vi "真正主程序.vi"() -> ()   [LabVIEW 2013]
doc: "该模板用于创建生产者／消费者模式的应用程序，以事件驱动的方式，生成队列中的项。如需通过响应事件实现代码的异步执行，同时不影响用户界面的响应速度，可考虑用该模式替代“用户界面事件处理器”模式。"
panel:
  in  "战斗失败":bool
  out "怪物血值":i32=380
  in  "战斗胜利":bool
  out "五个状态 2":enum16{"神不足", "逃跑", "初始化", "物品", "仙术", "攻击"}(ring)=enum."逃跑"
  in  "神值不够":bool
  in  "逃跑成功":bool
  out "沈欺霜 2":i32(slide) scale=0.0..200.0
  in  "龙蟠雕玉":cluster{"琉璃法珠":bool, "介绍框":bool, "剩余":dbl}
  in  "疾风术簇":T1
  in  "凝冰术簇":T2
  in  "火爪术簇":T3
  in  "普通攻击簇":T4
  out "集气攻击待机动作":bool
  in  "集气攻击簇":T5
  in  "怪物":bool=TRUE
  in  "确定按敌人攻击值钮":bool
  in  "怪兽 2":bool=TRUE
  in  "怪物状态":enum16{"初始化", "后退", "施法", "出击"}(ring)
  in  "枚举":enum16{"我方攻击", "敌人战斗", "时间条"}(ring)
  in  "主控":enum16{"我方攻击", "敌方攻击", "时间条", ""}(ring)
  out "怪物行走":i32(slide)=64 scale=0.0..100.0
  out "人物行走":i32(slide)=105 scale=0.0..100.0
  in  "待机":bool
  out "神":i32(slide)=150 scale=0.0..200.0
  out "沈欺霜":i32(slide)=150 scale=0.0..200.0
  in  "琉璃法珠簇":cluster{"琉璃法珠":bool, "介绍框":bool, "剩余":dbl}
  in  "仙术簇":T6={"火爪术"=TRUE, "凝冰术"=FALSE, "疾风术"=FALSE, "仙术中的放弃"=TRUE}
  in  "物品簇":cluster{"止血草":bool, "鼠儿果":bool, "物品中的放弃":bool}={"止血草"=FALSE, "鼠儿果"=FALSE, "物品中的放弃"=TRUE}
  in  "攻击簇":cluster{"普通攻击":bool, "集气攻击":bool, "攻击中的放弃":bool}={"普通攻击"=TRUE, "集气攻击"=FALSE, "攻击中的放弃"=FALSE}
  in  "逃跑":bool
  in  "物品":bool
  in  "仙术":bool
  in  "攻击":bool
  in  "五个状态":enum16{"逃跑", "初始化", "物品", "仙术", "攻击"}(ring)
  in  "怪兽":bool
  # "框图坐标\n207,421,460，498\n沈欺霜坐标\n800,388"
  # "剩余"
  # "个"
  # "剩余"
  # "个"
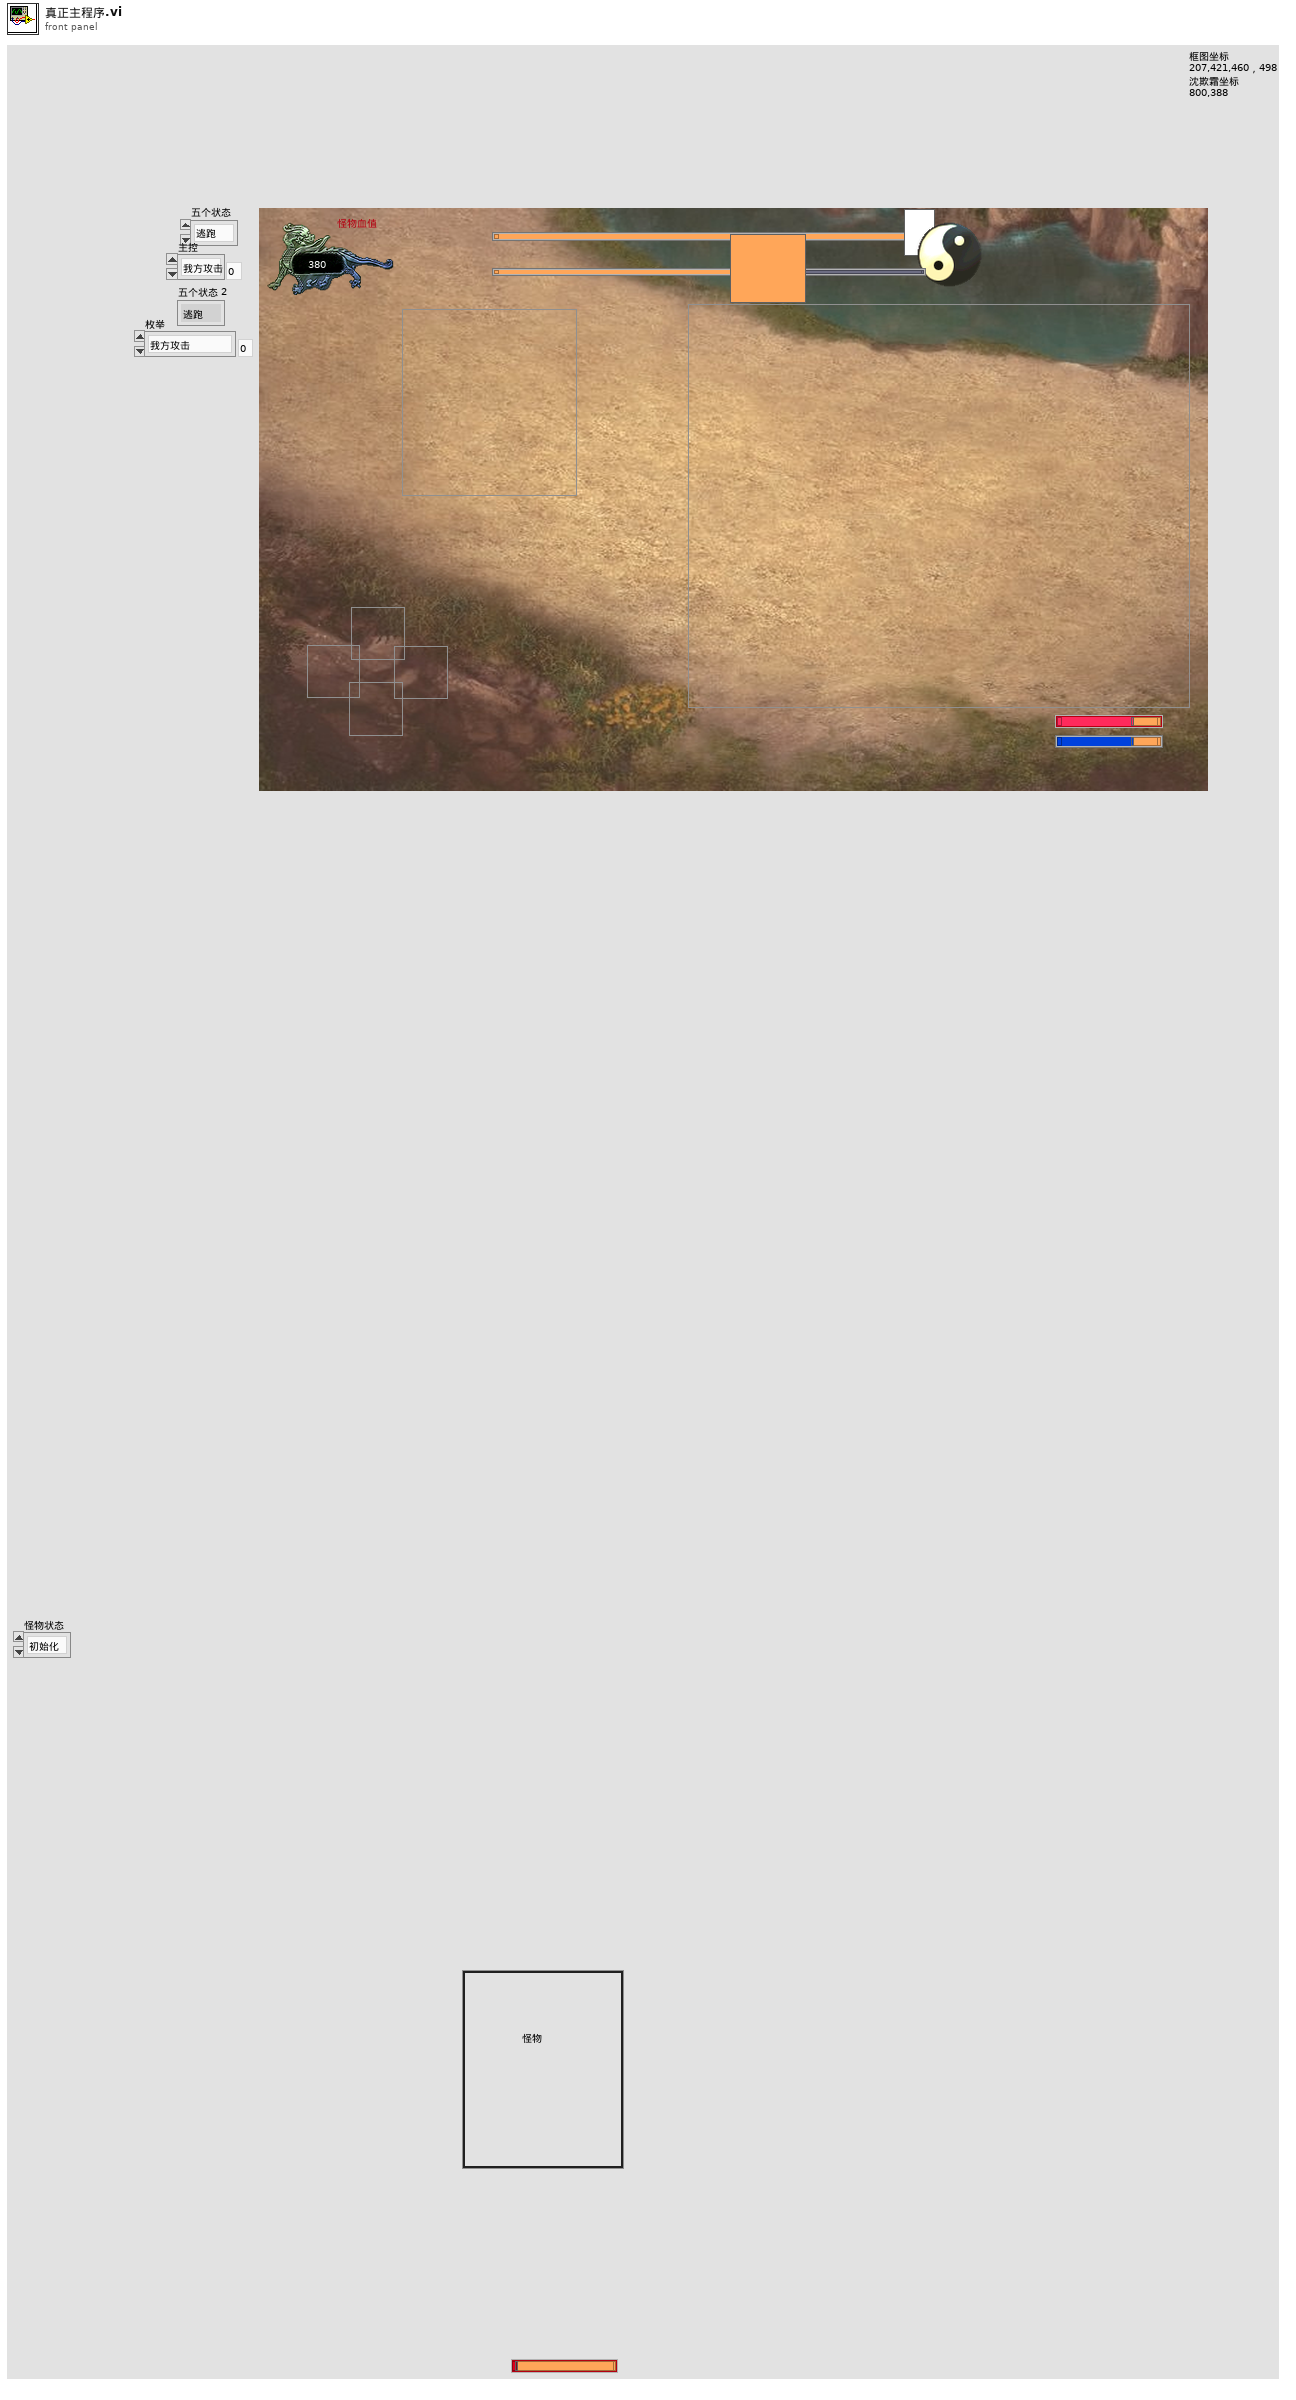
[diagram p1: front panel]
types:
  T1 = cluster{"确定按钮":bool, "确定按钮 2":bool, "确定按钮 3":bool, "确定按钮 4":bool, "确定按钮 5":bool, "确定按钮 6":bool, "确定按钮 7":bool, "确定按钮 8":bool, "确定按钮 9":bool, "确定按钮 10":bool, "确定按钮 11":bool, "确定按钮 12":bool, "确定按钮 13":bool, "确定按钮 14":bool, "确定按钮 15":bool}
  T2 = cluster{"确定按钮1":bool, "确定按钮 2":bool, "确定按钮 3":bool, "确定按钮 4":bool, "确定按钮 5":bool, "确定按钮 6":bool, "确定按钮 7":bool, "确定按钮 8":bool, "确定按钮 9":bool, "确定按钮 10":bool, "确定按钮 11":bool, "确定按钮 12":bool, "确定按钮 13":bool, "确定按钮 14":bool, "确定按钮 15":bool, bool}
  T3 = cluster{"4":bool, "5":bool, "6":bool, "7":bool, "8":bool, "1":bool, "2":bool, "3":bool, "9":bool, "10":bool, "11":bool, "12":bool, "13":bool, "14":bool, "15":bool, "确定按钮":bool}
  T4 = cluster{"1":bool, "2":bool, "3":bool, "4":bool, "5":bool, "6":bool, "7":bool, "8":bool, "9":bool, "减50":bool}
  T5 = cluster{"1":bool, "2":bool, "3":bool, "4":bool, "5":bool, "6":bool, "7":bool, "8":bool, "9":bool, "10":bool, "11":bool, "12":bool, "13":bool, "14":bool, "15":bool, "16":bool, "17":bool}
  T6 = cluster{"火爪术":bool, "凝冰术":bool, "疾风术":bool, "仙术中的放弃":bool}
  T7 = cluster{"1":bool, "2":bool, "3":bool, "4":bool, "5":bool, "6":bool, "7":bool, "8":bool, "9":bool}
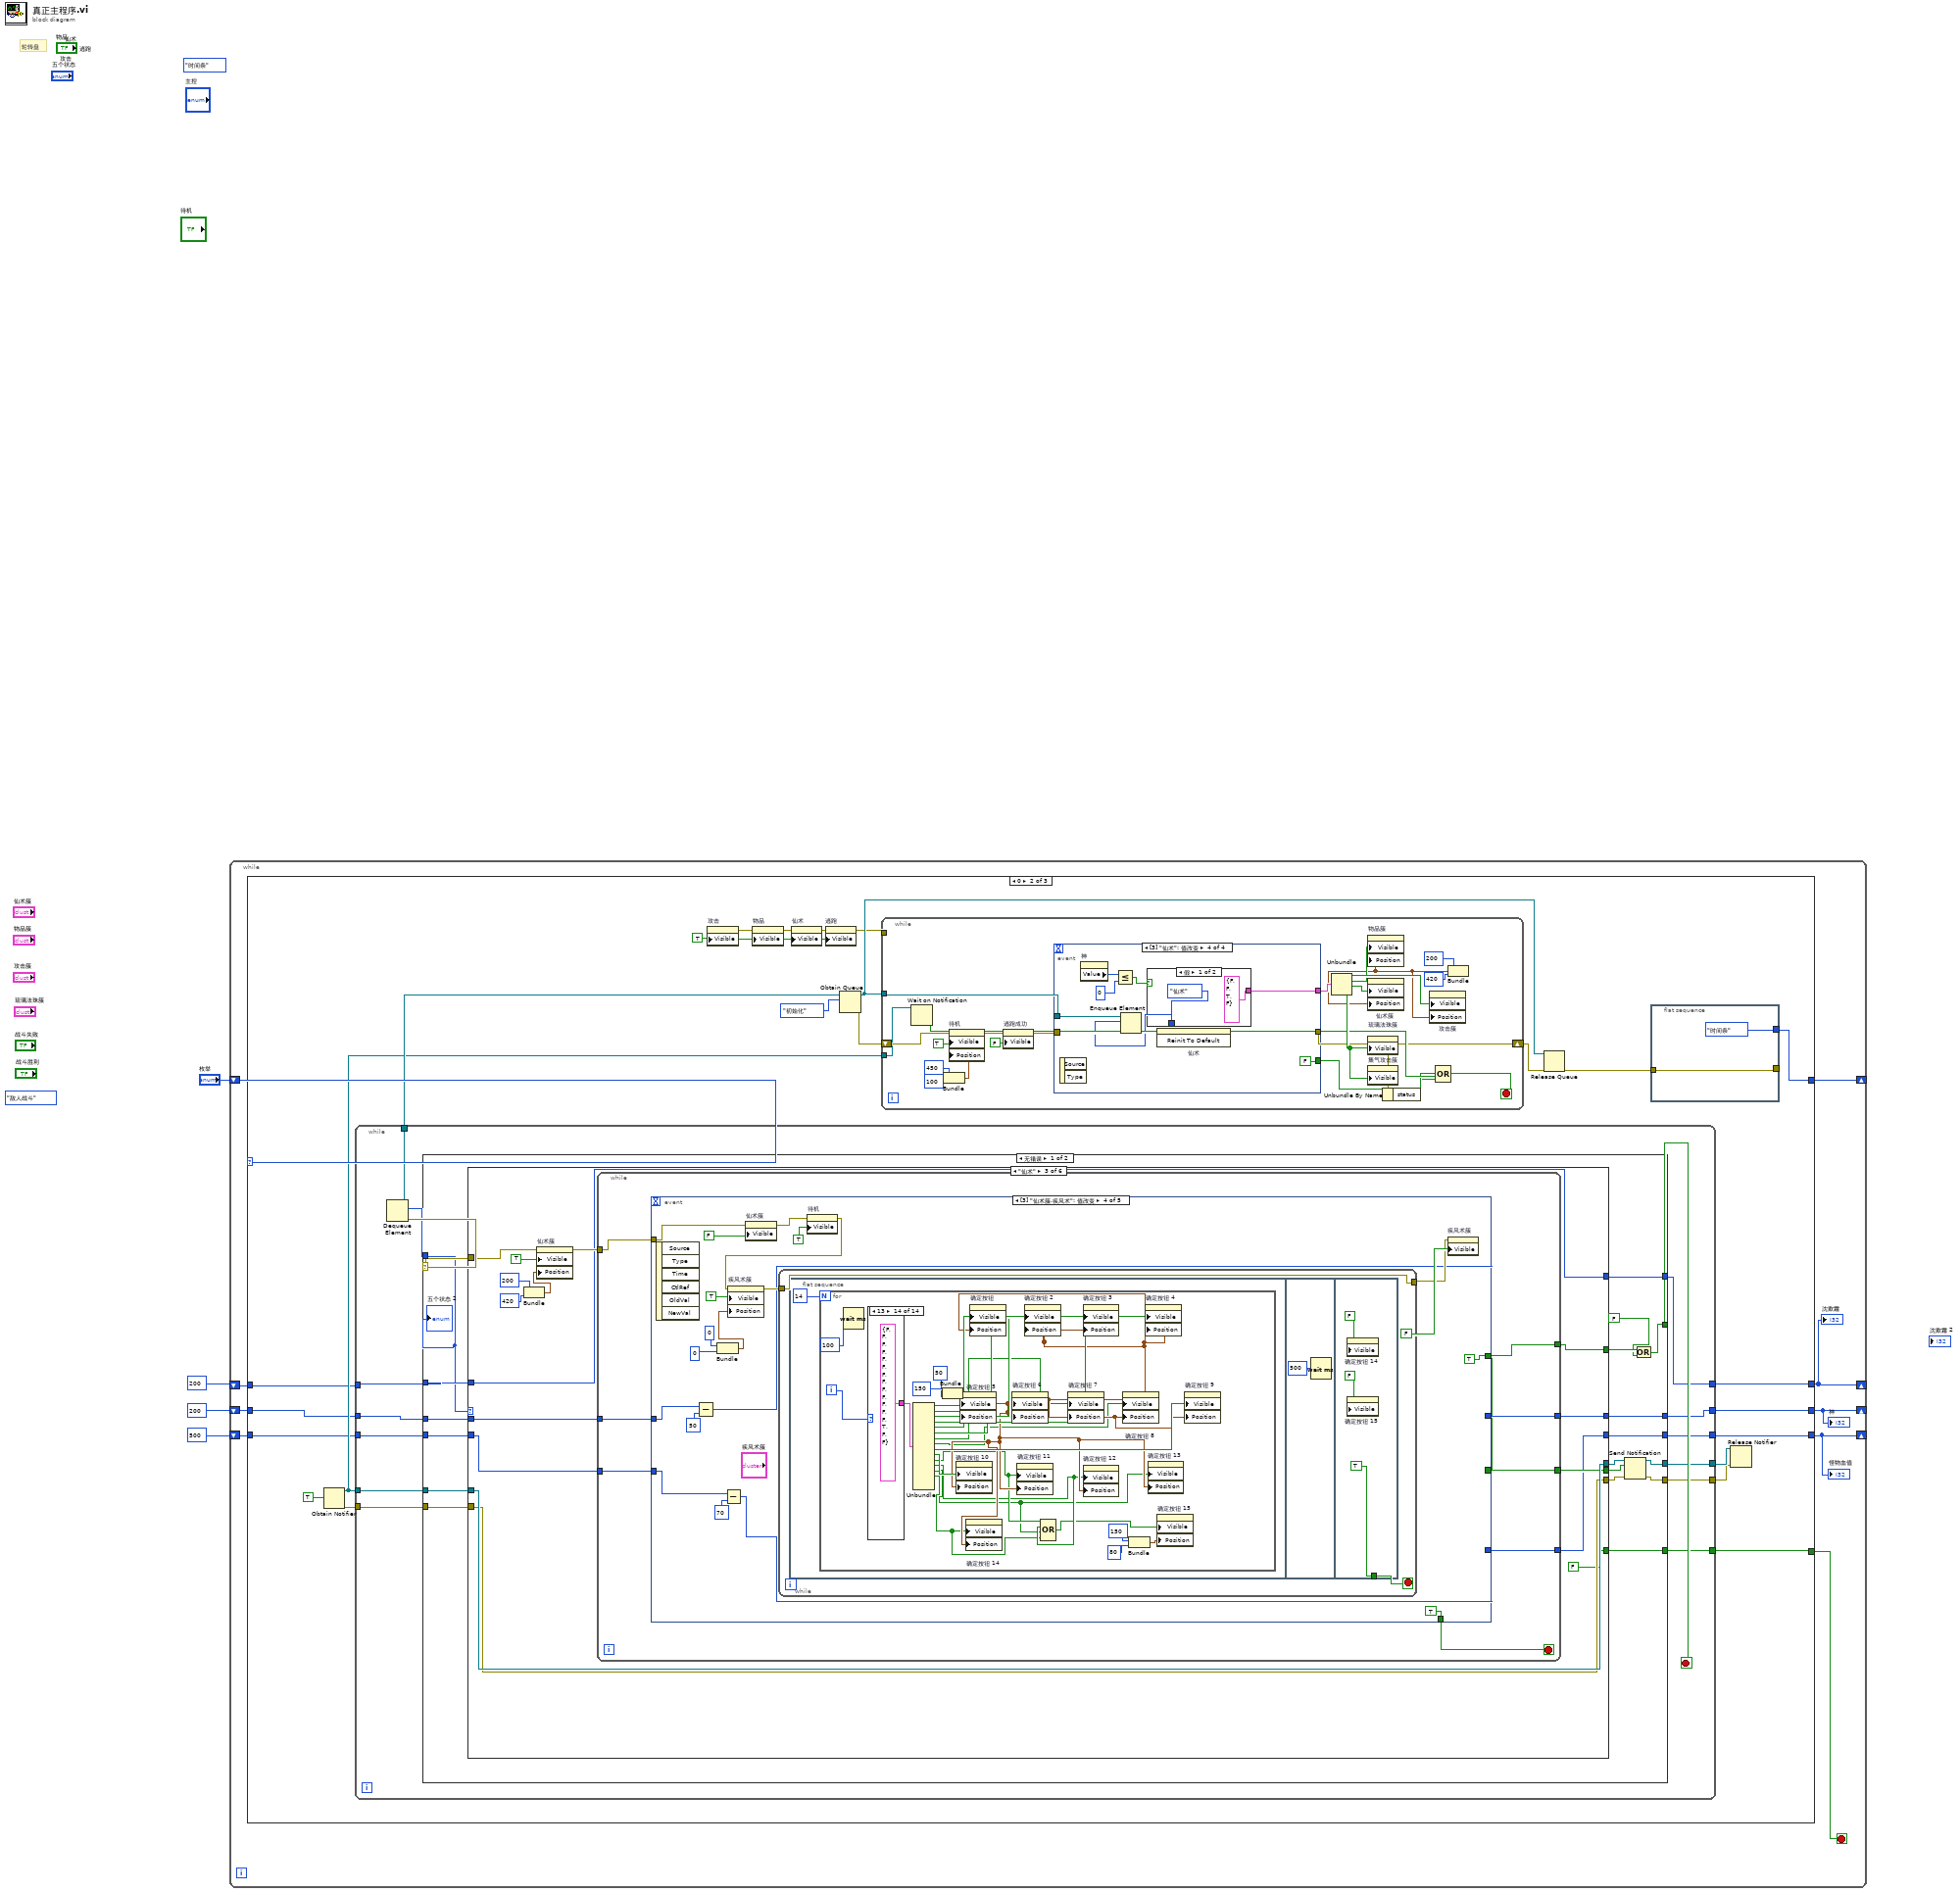
[diagram p0: block diagram]
diagram:
  (unwired) enum16{"我方攻击", "敌人战斗", "时间条"}."敌人战斗" ("枚举")
  (unwired) enum16{"我方攻击", "敌方攻击", "时间条", ""}."时间条" ("主控")
  # "轮转盘"
  n1 = while {
    shift-right: [w12] -> _
    shift-left: "枚举" -> [w13]
    shift-right: [w8] -> _
    shift-left: 200 -> [w11]
    shift-right: [w9] -> _
    shift-left: 200 -> [w10]
    shift-right: [w5] -> _
    shift-left: 500 -> [w7]
    stop <- w6 stop-if-true
    n2 = case shown="0" w13 {
      tunnel: [enum16{"我方攻击", "敌方攻击", "时间条", ""}."时间条" ("主控") w132 w790] -> w12
      tunnel: w11 -> [w22 w121 w784]
      tunnel: w10 -> [w21 w120 w789]
      tunnel: [w15 w119 w784] -> w8
      tunnel: [w21 w118 w789] -> w9
      tunnel: w7 -> [w20 w115 w786]
      tunnel: [w20 w114 w786] -> w5
      tunnel: [w17 w113 w785] -> w6
      frame 1 {
        w28 = FALSE
        n3 = Subtract(x=w22, y=50) -> (x-y=w16:i32)
        n4 = property on="攻击" class="Bool"("Visible"=w28) -> (error out=w27:errorcluster)  [unwired: 2 in, 1 out]
        n5 = property on="逃跑" class="Bool"(error in=w27, "Visible"=w28) -> (error out=w26:errorcluster)  [unwired: 1 in, 1 out]
        n6 = property on="物品" class="Bool"(error in=w26, "Visible"=w28) -> (error out=w25:errorcluster)  [unwired: 1 in, 1 out]
        n7 = property on="仙术" class="Bool"(error in=w25, "Visible"=w28) -> (error out=w24:errorcluster)  [unwired: 1 in, 1 out]
        n8 = while {
          shift-right: [w41] -> _
          shift-left: "怪物状态" -> [w43]
          tunnel: [w42] -> w14
          tunnel: w24 -> [_]
          stop <- w40 stop-if-true
          # "敌人攻击"
          n9 = case shown="\"后退\"" w43 {
            tunnel: [FALSE TRUE FALSE] -> w40
            tunnel: [w49 w61 w91] -> w42
            tunnel: [enum16{"初始化", "后退", "施法", "出击"}."出击" ("枚举") enum16{"初始化", "后退", "施法", "出击"}."初始化" ("枚举 2") enum16{"初始化", "后退", "施法", "出击"}."后退" ("枚举")] -> w41
            frame "初始化", Default {
              n10 = Bundle(550, 200) -> (w53:cluster{i32, i32})  [unwired: 1 in]
              n11 = Bundle(150, 100) -> (w54:cluster{i32, i32})  [unwired: 1 in]
              n12 = property on="怪兽" class="Bool"("Visible"=TRUE, "Position"=w54) -> (error out=w50:errorcluster)  [unwired: 2 in, 1 out]
              n13 = property on="怪兽 2" class="Bool"(error in=w50, "Visible"=FALSE, "Position"=w53) -> (error out=w49:errorcluster)  [unwired: 1 in, 1 out]
            }
            frame "后退" {
              n14 = property on="怪兽" class="Bool"("Visible"=FALSE) -> (error out=w59:errorcluster)  [unwired: 2 in, 1 out]
              n15 = for {
                N: 20 -> [_]
                tunnel: w59 -> [w76]
                tunnel: [w75] -> w63
                i -> [w73]
                n16 = Multiply(x=20, y=w73) -> (x*y=w77:i32)
                n17 = Subtract(x=550, y=w77) -> (x-y=w74:i32)
                n18 = Multiply(x=5, y=w73) -> (x*y=w71:i32)
                n19 = Wait (ms)(milliseconds to wait=u32 10 ("等待时间（毫秒）")) -> ()  [unwired: 1 out]
                n20 = Subtract(x=200, y=w71) -> (x-y=w69:i32)
                n21 = Bundle(w74, w69) -> (w80:cluster{i32, i32})  [unwired: 1 in]
                n22 = property on="怪兽 2" class="Bool"(error in=w76, "Visible"=TRUE, "Position"=w80) -> (error out=w75:errorcluster)  [unwired: 1 in, 1 out]
              }
              n23 = Bundle(150, 100) -> (w65:cluster{i32, i32})  [unwired: 1 in]
              n24 = property on="怪兽 2" class="Bool"(error in=w63, "Visible"=FALSE) -> (error out=w62:errorcluster)  [unwired: 1 in, 1 out]
              n25 = property on="怪兽" class="Bool"(error in=w62, "Visible"=TRUE, "Position"=w65) -> (error out=w61:errorcluster)  [unwired: 1 in, 1 out]
            }
            frame "出击" {
              n26 = for {
                N: 20 -> [_]
                tunnel: [w109] -> w94
                tunnel: [w102] -> w90
                tunnel: [w101] -> w86
                i -> [w107]
                n27 = Multiply(x=w107, y=20) -> (x*y=w101:i32)
                n28 = Add(x=150, y=w101) -> (x+y=w103:i32)
                n29 = Multiply(x=w107, y=5) -> (x*y=w106:i32)
                n30 = Wait (ms)(milliseconds to wait=u32 1 ("等待时间（毫秒）")) -> ()  [unwired: 1 out]
                n31 = Add(x=100, y=w106) -> (x+y=w102:i32)
                n32 = Bundle(w103, w102) -> (w111:cluster{i32, i32})  [unwired: 1 in]
                n33 = property on="怪兽" class="Bool"("Position"=w111) -> (error out=w109:errorcluster)  [unwired: 2 in, 1 out]
              }
              n34 = Subtract(x=w90, y=60) -> (x-y=w88:i32)
              n35 = Add(x=w86, y=300) -> (x+y=w85:i32)
              n36 = Bundle(w85, w88) -> (w84:cluster{i32, i32})  [unwired: 1 in]
              n37 = property on="确定按敌人攻击值钮" class="Bool"(error in=w94, "Visible"=TRUE, "Position"=w84) -> (error out=w93:errorcluster)  [unwired: 1 in, 1 out]
              n38 = flat-sequence {
                tunnel: w93 -> [w99]
                tunnel: [w99] -> _
                tunnel: [w99] -> w92
                frame #0 {
                  n39 = Wait (ms)(milliseconds to wait=500) -> ()  [unwired: 1 out]
                }
              }
              n40 = property on="确定按敌人攻击值钮" class="Bool"(error in=w92, "Visible"=FALSE) -> (error out=w91:errorcluster)  [unwired: 1 in, 1 out]
            }
          }
        }
        n41 = Less Or Equal?(x=w16, y=0) -> (x <= y?=w18:bool)
        n42 = case shown="假" w18 {
          tunnel: [FALSE w38] -> w17
          tunnel: w16 -> [w32 w39]
          tunnel: [w32 w39] -> w15
          tunnel: w14 -> [w31 w34]
          tunnel: [w31 w34] -> _
          frame False {
          }
          frame True {
            w38 = TRUE
            n43 = Bundle(200, 200) -> (w35:cluster{i32, i32})  [unwired: 1 in]
            n44 = property on="战斗失败" class="Bool"("Visible"=w38, "Position"=w35) -> ()  [unwired: 2 in, 2 out]
          }
        }
      }
      frame 0 {
        w123 = TRUE
        n45 = Obtain Notifier(notification data type=TRUE) -> (notifier out=w127:refnum<notifier>, error out=w128:errorcluster)  [unwired: 3 in, 1 out]
        n46 = property on="攻击" class="Bool"("Visible"=w123) -> (error out=w126:errorcluster)  [unwired: 2 in, 1 out]
        n47 = property on="物品" class="Bool"(error in=w126, "Visible"=w123) -> (error out=w125:errorcluster)  [unwired: 1 in, 1 out]
        n48 = property on="仙术" class="Bool"(error in=w125, "Visible"=w123) -> (error out=w124:errorcluster)  [unwired: 1 in, 1 out]
        n49 = property on="逃跑" class="Bool"(error in=w124, "Visible"=w123) -> (error out=w122:errorcluster)  [unwired: 1 in, 1 out]
        n50 = Obtain Queue(element data type=enum16{"神不足", "逃跑", "初始化", "物品", "仙术", "攻击"}."初始化" ("五个状态")) -> (queue out=w134:refnum<queue>, error out=w135:errorcluster)  [unwired: 4 in, 1 out]
        n51 = while {
          tunnel: w134 -> [w149]
          tunnel: w127 -> [w148]
          tunnel: [w147] -> w130
          tunnel: [w146] -> w129
          tunnel: w128 -> [w145]
          tunnel: w121 -> [w144]
          tunnel: w120 -> [w143]
          tunnel: [w142] -> w119
          tunnel: [w141] -> w118
          tunnel: w115 -> [w140]
          tunnel: [w139] -> w114
          tunnel: [w138] -> w113
          stop <- w150 stop-if-true
          n52 = Dequeue Element(queue=w149) -> (element=w151:enum16{"神不足", "逃跑", "初始化", "物品", "仙术", "攻击"}, error out=w152:errorcluster)  [unwired: 2 in, 2 out]
          n53 = case shown="无错误" w152 {
            selector: w152 -> [w171 _]
            tunnel: w151 -> [w156 _]
            tunnel: [w164 TRUE] -> w150
            tunnel: w144 -> [w170 w719]
            tunnel: [w169 w719] -> w142
            tunnel: w143 -> [w168 w718]
            tunnel: [w167 w718] -> w141
            tunnel: w148 -> [w163 w717]
            tunnel: [w157 w717] -> w147
            tunnel: [w158 w716] -> w146
            tunnel: w145 -> [w162 w716]
            tunnel: w140 -> [w155 w715]
            tunnel: [w154 w715] -> w139
            tunnel: [w153 TRUE] -> w138
            frame No Error {
              n54 = case shown="\"仙术\"" w156 {
                tunnel: w171 -> [_ w196 w366 w605 w690 _]
                tunnel: w170 -> [w179 w190 w364 w600 w689 w709]
                tunnel: [w179 w190 w364 w599 w689 w709] -> w169
                tunnel: w168 -> [w178 w189 w359 w594 w688 w708]
                tunnel: [w178 w189 w358 w593 w688 w708] -> w167
                tunnel: [FALSE w188 w363 w588 w683 FALSE] -> w166
                tunnel: w163 -> [w176 w187 w362 w590 w682 w705]
                tunnel: [w176 w185 w362 w590 w682 w705] -> w161
                tunnel: [w175 w183 w361 w589 w681 w704] -> w159
                tunnel: w162 -> [w175 w186 w361 w589 w681 w704]
                tunnel: [FALSE w184 w360 w588 TRUE FALSE] -> w160
                tunnel: w155 -> [w173 w182 w357 w587 w679 w696]
                tunnel: [w173 w181 w356 w587 w679 w696] -> w154
                tunnel: [FALSE FALSE FALSE FALSE TRUE FALSE] -> w153
                frame "初始化", Default {
                }
                frame "攻击" {
                  n55 = Bundle(200, 420) -> (w191:cluster{i32, i32})  [unwired: 1 in]
                  n56 = property on="攻击簇" class="Clust"(error in=w196, "Visible"=TRUE, "Position"=w191) -> (error out=w194:errorcluster)  [unwired: 1 in, 1 out]
                  n57 = while {
                    tunnel: w194 -> [w206]
                    tunnel: [w203] -> w188
                    tunnel: w187 -> [w202]
                    tunnel: w186 -> [w199]
                    tunnel: [w201] -> w185
                    tunnel: [w200] -> w184
                    tunnel: [w199] -> w183
                    tunnel: w182 -> [w198]
                    tunnel: [w197] -> w181
                    stop <- w207 stop-if-true
                    n58 = event shown="[3] \"攻击簇.普通攻击\": 值改变" {
                      selector: _ -> [_ _ _ _]
                      dyn-events: _ -> [_ _ _ _]
                      timeout: _ -> [_ _ _ _]
                      tunnel: [w210 w217 w299 w307] -> w205
                      tunnel: [FALSE TRUE TRUE TRUE] -> w207
                      tunnel: w206 -> [w210 w223 w299 w319]
                      tunnel: [w209 w215 w297 w305] -> w203
                      tunnel: w202 -> [w208 w216 w298 w304]
                      tunnel: [w208 w216 w298 w304] -> w201
                      tunnel: [w209 w215 w297 w305] -> w200
                      tunnel: w198 -> [_ w213 w296 w302]
                      tunnel: [_ w212 w296 w301] -> w197
                      event Timeout {
                        w209 = FALSE
                        n59 = event-data() -> ()  [unwired: 1 in, 3 out]
                      }
                      event "攻击簇.集气攻击": Value Change {
                        w215 = TRUE
                        w232 = TRUE ("可见")
                        n60 = event-data() -> ()  [unwired: 1 in, 6 out]
                        n61 = Bundle(450, 100) -> (w237:cluster{i32, i32})  [unwired: 1 in]
                        n62 = property on="待机" class="Bool"(error in=w223, "Visible"=FALSE) -> (error out=w224:errorcluster)  [unwired: 1 in, 1 out]
                        n63 = property on="攻击簇" class="Clust"(error in=w224, "Visible"=FALSE) -> (error out=w231:errorcluster)  [unwired: 1 in, 1 out]
                        n64 = property on="集气攻击待机动作" class="Bool"(error in=w231, "Position"=w237, "Visible"=w232) -> (error out=w240:errorcluster)  [unwired: 1 in, 1 out]
                        n65 = property on="集气攻击簇" class="Clust"(error in=w231, "Visible"=w232) -> (error out=w230:errorcluster)  [unwired: 1 in, 1 out]
                        n66 = Subtract(x=w213, y=100) -> (x-y=w212:i32)
                        n67 = for {
                          N: 20 -> [_]
                          shift-right: [w288] -> _
                          shift-left: _ -> [_]
                          tunnel: w240 -> [w289]
                          tunnel: [w289] -> w235
                          i -> [w290]
                          n68 = Quotient & Remainder(x=w290, y=2) -> (x-y*floor(x/y)=w292:i32)  [unwired: 1 out]
                          n69 = case shown="1" w292 {
                            tunnel: [TRUE FALSE] -> w288
                            frame 0, Default {
                            }
                            frame 1 {
                            }
                          }
                          "集气攻击待机动作" <- w288
                          n70 = Wait (ms)(milliseconds to wait=u32 100 ("等待时间（毫秒）")) -> ()  [unwired: 1 out]
                        }
                        n71 = while {
                          tunnel: w230 -> [w242]
                          tunnel: [w242] -> w229
                          stop <- w243 stop-if-true
                          n72 = flat-sequence {
                            tunnel: [TRUE] -> w243
                            frame #0 {
                              n73 = for {
                                N: 17 -> [_]
                                i -> [w256]
                                n74 = Wait (ms)(milliseconds to wait=100) -> ()  [unwired: 1 out]
                                n75 = case shown="0, 默认" w256 {
                                tunnel: [T5 {"1"=TRUE, "2"=FALSE, "3"=FALSE, "4"=FALSE, "5"=FALSE, "6"=FALSE, "7"=FALSE, "8"=FALSE, "9"=FALSE, "10"=FALSE, "11"=FALSE, "12"=FALSE, "13"=FALSE, "14"=FALSE, "15"=FALSE, "16"=FALSE, "17"=FALSE} ("簇") T5 {"1"=FALSE, "2"=TRUE, "3"=FALSE, "4"=FALSE, "5"=FALSE, "6"=FALSE, "7"=FALSE, "8"=FALSE, "9"=FALSE, "10"=FALSE, "11"=FALSE, "12"=FALSE, "13"=FALSE, "14"=FALSE, "15"=FALSE, "16"=FALSE, "17"=FALSE} ("簇") T5 {"1"=FALSE, "2"=FALSE, "3"=TRUE, "4"=FALSE, "5"=FALSE, "6"=FALSE, "7"=FALSE, "8"=FALSE, "9"=FALSE, "10"=FALSE, "11"=FALSE, "12"=FALSE, "13"=FALSE, "14"=FALSE, "15"=FALSE, "16"=FALSE, "17"=FALSE} ("簇") T5 {"1"=FALSE, "2"=FALSE, "3"=FALSE, "4"=TRUE, "5"=FALSE, "6"=FALSE, "7"=FALSE, "8"=FALSE, "9"=FALSE, "10"=FALSE, "11"=FALSE, "12"=FALSE, "13"=FALSE, "14"=FALSE, "15"=FALSE, "16"=FALSE, "17"=FALSE} ("簇") T5 {"1"=FALSE, "2"=FALSE, "3"=FALSE, "4"=FALSE, "5"=TRUE, "6"=FALSE, "7"=FALSE, "8"=FALSE, "9"=FALSE, "10"=FALSE, "11"=FALSE, "12"=FALSE, "13"=FALSE, "14"=FALSE, "15"=FALSE, "16"=FALSE, "17"=FALSE} ("簇") T5 {"1"=FALSE, "2"=FALSE, "3"=FALSE, "4"=FALSE, "5"=FALSE, "6"=TRUE, "7"=FALSE, "8"=FALSE, "9"=FALSE, "10"=FALSE, "11"=FALSE, "12"=FALSE, "13"=FALSE, "14"=FALSE, "15"=FALSE, "16"=FALSE, "17"=FALSE} ("簇") T5 {"1"=FALSE, "2"=FALSE, "3"=FALSE, "4"=FALSE, "5"=FALSE, "6"=FALSE, "7"=TRUE, "8"=FALSE, "9"=FALSE, "10"=FALSE, "11"=FALSE, "12"=FALSE, "13"=FALSE, "14"=FALSE, "15"=FALSE, "16"=FALSE, "17"=FALSE} ("簇") T5 {"1"=FALSE, "2"=FALSE, "3"=FALSE, "4"=FALSE, "5"=FALSE, "6"=FALSE, "7"=FALSE, "8"=TRUE, "9"=FALSE, "10"=FALSE, "11"=FALSE, "12"=FALSE, "13"=FALSE, "14"=FALSE, "15"=FALSE, "16"=FALSE, "17"=FALSE} ("簇") T5 {"1"=FALSE, "2"=FALSE, "3"=FALSE, "4"=FALSE, "5"=FALSE, "6"=FALSE, "7"=FALSE, "8"=FALSE, "9"=TRUE, "10"=FALSE, "11"=FALSE, "12"=FALSE, "13"=FALSE, "14"=FALSE, "15"=FALSE, "16"=FALSE, "17"=FALSE} ("簇") T5 {"1"=FALSE, "2"=FALSE, "3"=FALSE, "4"=FALSE, "5"=FALSE, "6"=FALSE, "7"=FALSE, "8"=FALSE, "9"=FALSE, "10"=TRUE, "11"=FALSE, "12"=FALSE, "13"=FALSE, "14"=FALSE, "15"=FALSE, "16"=FALSE, "17"=FALSE} ("簇") T5 {"1"=FALSE, "2"=FALSE, "3"=FALSE, "4"=FALSE, "5"=FALSE, "6"=FALSE, "7"=FALSE, "8"=FALSE, "9"=FALSE, "10"=FALSE, "11"=TRUE, "12"=FALSE, "13"=FALSE, "14"=FALSE, "15"=FALSE, "16"=FALSE, "17"=FALSE} ("簇") T5 {"1"=FALSE, "2"=FALSE, "3"=FALSE, "4"=FALSE, "5"=FALSE, "6"=FALSE, "7"=FALSE, "8"=FALSE, "9"=FALSE, "10"=FALSE, "11"=FALSE, "12"=TRUE, "13"=FALSE, "14"=FALSE, "15"=FALSE, "16"=FALSE, "17"=FALSE} ("簇") T5 {"1"=FALSE, "2"=FALSE, "3"=FALSE, "4"=FALSE, "5"=FALSE, "6"=FALSE, "7"=FALSE, "8"=FALSE, "9"=FALSE, "10"=FALSE, "11"=FALSE, "12"=FALSE, "13"=TRUE, "14"=FALSE, "15"=FALSE, "16"=FALSE, "17"=FALSE} ("簇") T5 {"1"=FALSE, "2"=FALSE, "3"=FALSE, "4"=FALSE, "5"=FALSE, "6"=FALSE, "7"=FALSE, "8"=FALSE, "9"=FALSE, "10"=FALSE, "11"=FALSE, "12"=FALSE, "13"=FALSE, "14"=TRUE, "15"=FALSE, "16"=FALSE, "17"=FALSE} ("簇") T5 {"1"=FALSE, "2"=FALSE, "3"=FALSE, "4"=FALSE, "5"=FALSE, "6"=FALSE, "7"=FALSE, "8"=FALSE, "9"=FALSE, "10"=FALSE, "11"=FALSE, "12"=FALSE, "13"=FALSE, "14"=FALSE, "15"=TRUE, "16"=FALSE, "17"=FALSE} ("簇") T5 {"1"=FALSE, "2"=FALSE, "3"=FALSE, "4"=FALSE, "5"=FALSE, "6"=FALSE, "7"=FALSE, "8"=FALSE, "9"=FALSE, "10"=FALSE, "11"=FALSE, "12"=FALSE, "13"=FALSE, "14"=FALSE, "15"=FALSE, "16"=TRUE, "17"=FALSE} ("簇") T5 {"1"=FALSE, "2"=FALSE, "3"=FALSE, "4"=FALSE, "5"=FALSE, "6"=FALSE, "7"=FALSE, "8"=FALSE, "9"=FALSE, "10"=FALSE, "11"=FALSE, "12"=FALSE, "13"=FALSE, "14"=FALSE, "15"=FALSE, "16"=FALSE, "17"=TRUE} ("簇")] -> w255
                                frame 0, Default {
                                }
                                frame 1 {
                                }
                                frame 2 {
                                }
                                frame 3 {
                                }
                                frame 4 {
                                }
                                frame 5 {
                                }
                                frame 6 {
                                }
                                frame 7 {
                                }
                                frame 8 {
                                }
                                frame 9 {
                                }
                                frame 10 {
                                }
                                frame 11 {
                                }
                                frame 12 {
                                }
                                frame 13 {
                                }
                                frame 14 {
                                }
                                frame 15 {
                                }
                                frame 16 {
                                }
                                }
                                n76 = Unbundle(w255) -> ("1"=w266:bool, "2"=w265:bool, "3"=w264:bool, "4"=w263:bool, "5"=w262:bool, "6"=w261:bool, "7"=w260:bool, "8"=w259:bool, "9"=w257:bool, "10"=w254:bool, "11"=w253:bool, "12"=w252:bool, "13"=w251:bool, "14"=w250:bool, "15"=w249:bool, "16"=w248:bool, "17"=w247:bool)
                                n77 = Bundle(50, -20) -> (w246:cluster{i32, i32})  [unwired: 1 in]
                                n78 = property on="10" class="Bool"("Visible"=w254, "Position"=w246) -> ()  [unwired: 2 in, 2 out]
                                n79 = property on="5" class="Bool"("Visible"=w262, "Position"=w246) -> ()  [unwired: 2 in, 2 out]
                                n80 = property on="1" class="Bool"("Visible"=w266, "Position"=w246) -> ()  [unwired: 2 in, 2 out]
                                n81 = property on="14" class="Bool"("Visible"=w250, "Position"=w246) -> ()  [unwired: 2 in, 2 out]
                                n82 = property on="6" class="Bool"("Visible"=w261, "Position"=w246) -> ()  [unwired: 2 in, 2 out]
                                n83 = property on="11" class="Bool"("Visible"=w253, "Position"=w246) -> ()  [unwired: 2 in, 2 out]
                                n84 = property on="2" class="Bool"("Visible"=w265, "Position"=w246) -> ()  [unwired: 2 in, 2 out]
                                n85 = property on="3" class="Bool"("Visible"=w264, "Position"=w246) -> ()  [unwired: 2 in, 2 out]
                                n86 = property on="7" class="Bool"("Visible"=w260, "Position"=w246) -> ()  [unwired: 2 in, 2 out]
                                n87 = property on="12" class="Bool"("Visible"=w252, "Position"=w246) -> ()  [unwired: 2 in, 2 out]
                                n88 = property on="15" class="Bool"("Visible"=w249, "Position"=w246) -> ()  [unwired: 2 in, 2 out]
                                n89 = property on="4" class="Bool"("Visible"=w263, "Position"=w246) -> ()  [unwired: 2 in, 2 out]
                                n90 = property on="13" class="Bool"("Visible"=w251, "Position"=w246) -> ()  [unwired: 2 in, 2 out]
                                n91 = property on="8" class="Bool"("Visible"=w259, "Position"=w246) -> ()  [unwired: 2 in, 2 out]
                                n92 = property on="17" class="Bool"("Visible"=w247, "Position"=w246) -> ()  [unwired: 2 in, 2 out]
                                n93 = property on="16" class="Bool"("Visible"=w248, "Position"=w246) -> ()  [unwired: 2 in, 2 out]
                                n94 = property on="9" class="Bool"("Visible"=w257, "Position"=w246) -> ()  [unwired: 2 in, 2 out]
                              }
                            }
                            frame #1 {
                              n95 = Wait (ms)(milliseconds to wait=500) -> ()  [unwired: 1 out]
                            }
                            frame #2 {
                              n96 = property on="17" class="Bool"("Visible"=FALSE) -> ()  [unwired: 2 in, 2 out]
                            }
                          }
                        }
                        n97 = property on="集气攻击待机动作" class="Bool"(error in=w235, "Visible"=FALSE) -> (error out=w227:errorcluster)  [unwired: 1 in, 1 out]
                        n98 = property on="集气攻击簇" class="Clust"(error in=w229, "Visible"=FALSE) -> (error out=w226:errorcluster)  [unwired: 1 in, 1 out]
                        n99 = Merge Errors(w227, w226) -> (w218:errorcluster)
                        n100 = Bundle(450, 100) -> (w220:cluster{i32, i32})  [unwired: 1 in]
                        n101 = property on="待机" class="Bool"(error in=w218, "Visible"=TRUE, "Position"=w220) -> (error out=w217:errorcluster)  [unwired: 1 in, 1 out]
                      }
                      event "攻击簇.攻击中的放弃": Value Change {
                        w297 = FALSE
                        n102 = event-data() -> ()  [unwired: 1 in, 6 out]
                      }
                      event "攻击簇.普通攻击": Value Change {
                        w305 = TRUE
                        n103 = event-data() -> ()  [unwired: 1 in, 6 out]
                        n104 = Bundle(0, 0) -> (w314:cluster{i32, i32})  [unwired: 1 in]
                        n105 = property on="待机" class="Bool"(error in=w319, "Visible"=FALSE) -> (error out=w318:errorcluster)  [unwired: 1 in, 1 out]
                        n106 = property on="攻击簇" class="Clust"(error in=w318, "Visible"=FALSE) -> (error out=w312:errorcluster)  [unwired: 1 in, 1 out]
                        n107 = property on="普通攻击簇" class="Clust"(error in=w312, "Visible"=TRUE, "Position"=w314) -> (error out=w313:errorcluster)  [unwired: 1 in, 1 out]
                        n108 = Subtract(x=w302, y=50) -> (x-y=w301:i32)
                        n109 = while {
                          tunnel: w313 -> [w322]
                          tunnel: [w322] -> w310
                          stop <- w323 stop-if-true
                          n110 = flat-sequence {
                            tunnel: [TRUE] -> w323
                            frame #0 {
                              n111 = for {
                                N: 9 -> [_]
                                i -> [w331]
                                n112 = Wait (ms)(milliseconds to wait=120) -> ()  [unwired: 1 out]
                                n113 = case shown="0, 默认" w331 {
                                tunnel: [T7 {"1"=TRUE, "2"=FALSE, "3"=FALSE, "4"=FALSE, "5"=FALSE, "6"=FALSE, "7"=FALSE, "8"=FALSE, "9"=FALSE} ("簇") T7 {"1"=FALSE, "2"=TRUE, "3"=FALSE, "4"=FALSE, "5"=FALSE, "6"=FALSE, "7"=FALSE, "8"=FALSE, "9"=FALSE} ("簇") T7 {"1"=FALSE, "2"=FALSE, "3"=TRUE, "4"=FALSE, "5"=FALSE, "6"=FALSE, "7"=FALSE, "8"=FALSE, "9"=FALSE} ("簇") T7 {"1"=FALSE, "2"=FALSE, "3"=FALSE, "4"=TRUE, "5"=FALSE, "6"=FALSE, "7"=FALSE, "8"=FALSE, "9"=FALSE} ("簇") T7 {"1"=FALSE, "2"=FALSE, "3"=FALSE, "4"=FALSE, "5"=TRUE, "6"=FALSE, "7"=FALSE, "8"=FALSE, "9"=FALSE} ("簇") T7 {"1"=FALSE, "2"=FALSE, "3"=FALSE, "4"=FALSE, "5"=FALSE, "6"=TRUE, "7"=FALSE, "8"=FALSE, "9"=FALSE} ("簇") T7 {"1"=FALSE, "2"=FALSE, "3"=FALSE, "4"=FALSE, "5"=FALSE, "6"=FALSE, "7"=TRUE, "8"=FALSE, "9"=FALSE} ("簇") T7 {"1"=FALSE, "2"=FALSE, "3"=FALSE, "4"=FALSE, "5"=FALSE, "6"=FALSE, "7"=FALSE, "8"=TRUE, "9"=FALSE} ("簇") T7 {"1"=FALSE, "2"=FALSE, "3"=FALSE, "4"=FALSE, "5"=FALSE, "6"=FALSE, "7"=FALSE, "8"=FALSE, "9"=TRUE} ("簇")] -> w330
                                frame 0, Default {
                                }
                                frame 1 {
                                }
                                frame 2 {
                                }
                                frame 3 {
                                }
                                frame 4 {
                                }
                                frame 5 {
                                }
                                frame 6 {
                                }
                                frame 7 {
                                }
                                frame 8 {
                                }
                                }
                                n114 = Bundle(0, 10) -> (w329:cluster{i32, i32})  [unwired: 1 in]
                                n115 = Unbundle(w330) -> ("1"=w341:bool, "2"=w340:bool, "3"=w339:bool, "4"=w338:bool, "5"=w337:bool, "6"=w336:bool, "7"=w335:bool, "8"=w334:bool, "9"=w328:bool)
                                n116 = property on="5" class="Bool"("Visible"=w337, "Position"=w329) -> ()  [unwired: 2 in, 2 out]
                                n117 = property on="1" class="Bool"("Visible"=w341, "Position"=w329) -> ()  [unwired: 2 in, 2 out]
                                n118 = property on="6" class="Bool"("Visible"=w336, "Position"=w329) -> ()  [unwired: 2 in, 2 out]
                                n119 = property on="2" class="Bool"("Visible"=w340, "Position"=w329) -> ()  [unwired: 2 in, 2 out]
                                n120 = property on="7" class="Bool"("Visible"=w335, "Position"=w329) -> ()  [unwired: 2 in, 2 out]
                                n121 = property on="3" class="Bool"("Visible"=w339, "Position"=w329) -> ()  [unwired: 2 in, 2 out]
                                n122 = property on="8" class="Bool"("Visible"=w334, "Position"=w329) -> ()  [unwired: 2 in, 2 out]
                                n123 = property on="4" class="Bool"("Visible"=w338, "Position"=w329) -> ()  [unwired: 2 in, 2 out]
                                n124 = Bundle(100, 100) -> (w325:cluster{i32, i32})  [unwired: 1 in]
                                n125 = property on="9" class="Bool"("Visible"=w328, "Position"=w329) -> ()  [unwired: 2 in, 2 out]
                                n126 = property on="减50" class="Bool"("Visible"=w328, "Position"=w325) -> ()  [unwired: 2 in, 2 out]
                              }
                            }
                            frame #1 {
                              n127 = Wait (ms)(milliseconds to wait=500) -> ()  [unwired: 1 out]
                            }
                            frame #2 {
                              w354 = FALSE
                              n128 = property on="9" class="Bool"("Visible"=w354) -> ()  [unwired: 2 in, 2 out]
                              n129 = property on="减50" class="Bool"("Visible"=w354) -> ()  [unwired: 2 in, 2 out]
                            }
                          }
                        }
                        n130 = property on="普通攻击簇" class="Clust"(error in=w310, "Visible"=FALSE) -> (error out=w309:errorcluster)  [unwired: 1 in, 1 out]
                        n131 = property on="待机" class="Bool"(error in=w309, "Visible"=TRUE) -> (error out=w307:errorcluster)  [unwired: 1 in, 1 out]
                      }
                    }
                    n132 = property on="攻击簇" class="Clust"(error in=w205, "Visible"=FALSE) -> ()  [unwired: 1 in, 2 out]
                  }
                }
                frame "仙术" {
                  n133 = Bundle(200, 420) -> (w367:cluster{i32, i32})  [unwired: 1 in]
                  n134 = property on="仙术簇" class="Clust"(error in=w366, "Visible"=TRUE, "Position"=w367) -> (error out=w365:errorcluster)  [unwired: 1 in, 1 out]
                  n135 = while {
                    tunnel: w365 -> [w378]
                    tunnel: [w376] -> w363
                    tunnel: [w375] -> w360
                    tunnel: w359 -> [w374]
                    tunnel: [w373] -> w358
                    tunnel: w357 -> [w372]
                    tunnel: [w371] -> w356
                    stop <- w377 stop-if-true
                    n136 = event shown="[3] \"仙术簇.疾风术\": 值改变" {
                      selector: _ -> [_ _ _ _ _]
                      dyn-events: _ -> [_ _ _ _ _]
                      timeout: _ -> [_ _ _ _ _]
                      tunnel: w378 -> [_ w397 w463 w529 w583]
                      tunnel: [FALSE TRUE TRUE TRUE TRUE] -> w377
                      tunnel: [w381 w389 w455 w521 w582] -> w376
                      tunnel: [w381 w389 w455 w521 w582] -> w375
                      tunnel: w374 -> [w380 w387 w453 w519 w581]
                      tunnel: [w380 w386 w452 w518 w581] -> w373
                      tunnel: w372 -> [w379 w384 w450 w516 w580]
                      tunnel: [w379 w383 w449 w515 w580] -> w371
                      event Timeout {
                        w381 = FALSE
                        n137 = event-data() -> ()  [unwired: 1 in, 3 out]
                      }
                      event "仙术簇.火爪术": Value Change {
                        w389 = TRUE
                        n138 = event-data() -> ()  [unwired: 1 in, 6 out]
                        n139 = Subtract(x=w387, y=50) -> (x-y=w386:i32)
                        n140 = Bundle(0, 0) -> (w394:cluster{i32, i32})  [unwired: 1 in]
                        n141 = Subtract(x=w384, y=70) -> (x-y=w383:i32)
                        n142 = property on="仙术簇" class="Clust"(error in=w397, "Visible"=FALSE) -> (error out=w400:errorcluster)  [unwired: 1 in, 1 out]
                        n143 = property on="待机" class="Bool"(error in=w400, "Visible"=TRUE) -> (error out=w398:errorcluster)  [unwired: 1 in, 1 out]
                        n144 = property on="火爪术簇" class="Clust"(error in=w398, "Visible"=TRUE, "Position"=w394) -> (error out=w393:errorcluster)  [unwired: 1 in, 1 out]
                        n145 = while {
                          tunnel: w393 -> [w403]
                          tunnel: [w403] -> w392
                          stop <- w404 stop-if-true
                          n146 = flat-sequence {
                            tunnel: [TRUE] -> w404
                            frame #0 {
                              n147 = for {
                                N: 15 -> [_]
                                i -> [w416]
                                n148 = Wait (ms)(milliseconds to wait=100) -> ()  [unwired: 1 out]
                                n149 = case shown="2" w416 {
                                tunnel: [T3 {"4"=TRUE, "5"=FALSE, "6"=FALSE, "7"=FALSE, "8"=FALSE, "1"=FALSE, "2"=FALSE, "3"=FALSE, "9"=FALSE, "10"=FALSE, "11"=FALSE, "12"=FALSE, "13"=FALSE, "14"=FALSE, "15"=FALSE, "确定按钮"=FALSE} ("簇") T3 {"4"=FALSE, "5"=TRUE, "6"=FALSE, "7"=FALSE, "8"=FALSE, "1"=FALSE, "2"=FALSE, "3"=FALSE, "9"=FALSE, "10"=FALSE, "11"=FALSE, "12"=FALSE, "13"=FALSE, "14"=FALSE, "15"=FALSE, "确定按钮"=FALSE} ("簇") T3 {"4"=FALSE, "5"=FALSE, "6"=TRUE, "7"=FALSE, "8"=FALSE, "1"=FALSE, "2"=FALSE, "3"=FALSE, "9"=FALSE, "10"=FALSE, "11"=FALSE, "12"=FALSE, "13"=FALSE, "14"=FALSE, "15"=FALSE, "确定按钮"=FALSE} ("簇") T3 {"4"=FALSE, "5"=FALSE, "6"=FALSE, "7"=TRUE, "8"=FALSE, "1"=FALSE, "2"=FALSE, "3"=FALSE, "9"=FALSE, "10"=FALSE, "11"=FALSE, "12"=FALSE, "13"=FALSE, "14"=FALSE, "15"=FALSE, "确定按钮"=FALSE} ("簇") T3 {"4"=FALSE, "5"=FALSE, "6"=FALSE, "7"=FALSE, "8"=TRUE, "1"=FALSE, "2"=FALSE, "3"=FALSE, "9"=FALSE, "10"=FALSE, "11"=FALSE, "12"=FALSE, "13"=FALSE, "14"=FALSE, "15"=FALSE, "确定按钮"=FALSE} ("簇") T3 {"4"=FALSE, "5"=FALSE, "6"=FALSE, "7"=FALSE, "8"=FALSE, "1"=TRUE, "2"=FALSE, "3"=FALSE, "9"=FALSE, "10"=FALSE, "11"=FALSE, "12"=FALSE, "13"=FALSE, "14"=FALSE, "15"=FALSE, "确定按钮"=FALSE} ("簇") T3 {"4"=FALSE, "5"=FALSE, "6"=FALSE, "7"=FALSE, "8"=FALSE, "1"=FALSE, "2"=TRUE, "3"=FALSE, "9"=FALSE, "10"=FALSE, "11"=FALSE, "12"=FALSE, "13"=FALSE, "14"=FALSE, "15"=FALSE, "确定按钮"=FALSE} ("簇") T3 {"4"=FALSE, "5"=FALSE, "6"=FALSE, "7"=FALSE, "8"=FALSE, "1"=FALSE, "2"=FALSE, "3"=TRUE, "9"=FALSE, "10"=FALSE, "11"=FALSE, "12"=FALSE, "13"=FALSE, "14"=FALSE, "15"=FALSE, "确定按钮"=FALSE} ("簇") T3 {"4"=FALSE, "5"=FALSE, "6"=FALSE, "7"=FALSE, "8"=FALSE, "1"=FALSE, "2"=FALSE, "3"=FALSE, "9"=TRUE, "10"=FALSE, "11"=FALSE, "12"=FALSE, "13"=FALSE, "14"=FALSE, "15"=FALSE, "确定按钮"=FALSE} ("簇") T3 {"4"=FALSE, "5"=FALSE, "6"=FALSE, "7"=FALSE, "8"=FALSE, "1"=FALSE, "2"=FALSE, "3"=FALSE, "9"=FALSE, "10"=TRUE, "11"=FALSE, "12"=FALSE, "13"=FALSE, "14"=FALSE, "15"=FALSE, "确定按钮"=FALSE} ("簇") T3 {"4"=FALSE, "5"=FALSE, "6"=FALSE, "7"=FALSE, "8"=FALSE, "1"=FALSE, "2"=FALSE, "3"=FALSE, "9"=FALSE, "10"=FALSE, "11"=TRUE, "12"=FALSE, "13"=FALSE, "14"=FALSE, "15"=FALSE, "确定按钮"=FALSE} ("簇") T3 {"4"=FALSE, "5"=FALSE, "6"=FALSE, "7"=FALSE, "8"=FALSE, "1"=FALSE, "2"=FALSE, "3"=FALSE, "9"=FALSE, "10"=FALSE, "11"=FALSE, "12"=TRUE, "13"=FALSE, "14"=FALSE, "15"=FALSE, "确定按钮"=FALSE} ("簇") T3 {"4"=FALSE, "5"=FALSE, "6"=FALSE, "7"=FALSE, "8"=FALSE, "1"=FALSE, "2"=FALSE, "3"=FALSE, "9"=FALSE, "10"=FALSE, "11"=FALSE, "12"=FALSE, "13"=TRUE, "14"=FALSE, "15"=FALSE, "确定按钮"=FALSE} ("簇") T3 {"4"=FALSE, "5"=FALSE, "6"=FALSE, "7"=FALSE, "8"=FALSE, "1"=FALSE, "2"=FALSE, "3"=FALSE, "9"=FALSE, "10"=FALSE, "11"=FALSE, "12"=FALSE, "13"=FALSE, "14"=TRUE, "15"=FALSE, "确定按钮"=FALSE} ("簇") T3 {"4"=FALSE, "5"=FALSE, "6"=FALSE, "7"=FALSE, "8"=FALSE, "1"=FALSE, "2"=FALSE, "3"=FALSE, "9"=FALSE, "10"=FALSE, "11"=FALSE, "12"=FALSE, "13"=FALSE, "14"=FALSE, "15"=TRUE, "确定按钮"=FALSE} ("簇")] -> w415
                                frame 0, Default {
                                }
                                frame 1 {
                                }
                                frame 2 {
                                }
                                frame 3 {
                                }
                                frame 4 {
                                }
                                frame 5 {
                                }
                                frame 6 {
                                }
                                frame 7 {
                                }
                                frame 8 {
                                }
                                frame 9 {
                                }
                                frame 10 {
                                }
                                frame 11 {
                                }
                                frame 12 {
                                }
                                frame 13 {
                                }
                                frame 14 {
                                }
                                }
                                n150 = Unbundle(w415) -> ("4"=w428:bool, "5"=w427:bool, "6"=w426:bool, "7"=w425:bool, "8"=w424:bool, "1"=w423:bool, "2"=w411:bool, "3"=w410:bool, "9"=w420:bool, "10"=w419:bool, "11"=w414:bool, "12"=w418:bool, "13"=w408:bool, "14"=w409:bool, "15"=w406:bool)  [unwired: 1 out]